vi "FlexMag - 23-03-2023.vi"() -> ()   [LabVIEW 2018] (continued)
          tunnel: [w8156 w8268 w8304 w8346 w8389 w8424 w8458 w8492] -> w8125
          frame 0, Default {
            n4720 = stacked-sequence {
              seq-local: [w8166 _] -> [_ w8224]
              seq-local: [w8165 _] -> [_ w8222]
              tunnel: w8159 -> [w8175 _]
              tunnel: w8158 -> [w8174 _]
              tunnel: [_ w8226] -> w8157
              tunnel: [_ w8225] -> w8156
              frame #0 {
                # "Address"
                # "Address"
                n4721 = Concatenate Strings("002" ("write buffer"), "00" ("string"), "309" ("string"), "02" ("string"), "=?" ("string")) -> (w8184:string)
                n4722 = String To Byte Array(string=w8184) -> (unsigned byte array=w8189:u8[])
                n4723 = for {
                  tunnel: w8189 -> [w8221] mode=indexing
                  shift-right: [w8219] -> w8191
                  shift-left: u8 0 -> [w8220]
                  n4724 = Add(x=w8221, y=w8220) -> (x+y=w8219:u8)
                }
                n4725 = Number To Decimal String(number=w8191) -> (decimal integer string=w8186:string)  [unwired: 1 in]
                n4726 = String Length(string=w8186) -> (length=w8187:i32)
                n4727 = case shown="3" w8187 {
                  tunnel: w8186 -> [_ w8214 w8217 w8218]
                  tunnel: ["" w8212 w8215 w8218] -> w8185
                  frame 0, Default {
                  }
                  frame 1 {
                    n4728 = Concatenate Strings("00" ("string"), w8214) -> (w8212:string)
                  }
                  frame 2 {
                    n4729 = Concatenate Strings("0" ("string"), w8217) -> (w8215:string)
                  }
                  frame 3 {
                  }
                }
                n4730 = Concatenate Strings(w8184, w8185, "\r") -> (w8176:string)
                n4731 = VISA Write(VISA resource name=w8175, write buffer=w8176, error in (no error)=w8174) -> (VISA resource name out=w8179:refnum<visa-resource-name>, error out=w8178:errorcluster)  [unwired: 1 out]
                n4732 = stacked-sequence {
                  tunnel: [w8210] -> w8181
                  tunnel: w8179 -> [w8210]
                  tunnel: [w8209] -> w8180
                  tunnel: w8178 -> [w8209]
                  frame #0 {
                    n4733 = Wait (ms)(milliseconds to wait=u32 100) -> ()  [unwired: 1 out]
                  }
                }
                n4734 = property class="Instr"(reference=w8181, error in=w8180) -> (reference out=w8183:refnum<visa-resource-name>, error out=w8182:errorcluster, "Serial Settings:Number of Bytes at Serial Port"=w8177:u32)
                n4735 = VISA Read(VISA resource name=w8183, byte count=w8177, error in (no error)=w8182) -> (VISA resource name out=w8166:refnum<visa-resource-name>, read buffer=w8160:string, error out=w8165:errorcluster)  [unwired: 1 out]
                n4736 = String Length(string=w8160) -> (length=w8173:i32)
                n4737 = Not Equal To 0?(x=w8173) -> (x != 0?=w8164:bool)
                n4738 = feedback #142() -> (w8162:bool)  [unwired: 1 in]
                n4739 = Concatenate Strings("002" ("regular expression"), "1030906" ("regular expression")) -> (w8172:string)
                n4740 = case shown="False" w8164 {
                  tunnel: [FALSE w8201] -> w8161
                  tunnel: [TRUE FALSE] -> w8163
                  tunnel: w8162 -> [_ w8199]
                  frame False {
                  }
                  frame True {
                    n4741 = call "Elapsed Time37"("Reset"=w8199) -> ("Elapsed Time (s)"=w8202:dbl)  [unwired: 11 in, 7 out]
                    n4742 = Greater?(x=w8202, y=5.0) -> (0:w8201:bool)
                  }
                }
                "tp1 com" <- w8161
                n4743 = feedback-in #142(w8163) -> ()
                n4744 = Match Pattern(string=w8160, regular expression=w8172) -> (after substring=w8167:string)  [unwired: 4 out]
                n4745 = String Length(string=w8167) -> (length=w8169:i32)
                n4746 = Not Equal To 0?(x=w8169) -> (x != 0?=w8168:bool)
                n4747 = case shown="True" w8168 {
                  tunnel: w8167 -> [_ w8204]
                  frame False {
                  }
                  frame True {
                    n4748 = String Subset(string=w8204, length (rest)=6 ("length (rest)")) -> (substring=w8206:string)  [unwired: 1 out]
                    n4749 = Decimal String To Number(string=w8206) -> (number=→"Tp1 speed gui":i32)  [unwired: 3 out]
                    "tp1 readout" <- w8204
                  }
                }
              }
              frame #1 {
                # "Address"
                # "Address"
                n4750 = Concatenate Strings("002" ("write buffer"), "00" ("string"), "307" ("string"), "02" ("string"), "=?" ("string")) -> (w8239:string)
                n4751 = String To Byte Array(string=w8239) -> (unsigned byte array=w8244:u8[])
                n4752 = for {
                  tunnel: w8244 -> [w8265] mode=indexing
                  shift-right: [w8263] -> w8246
                  shift-left: u8 0 -> [w8264]
                  n4753 = Add(x=w8265, y=w8264) -> (x+y=w8263:u8)
                }
                n4754 = Number To Decimal String(number=w8246) -> (decimal integer string=w8241:string)  [unwired: 1 in]
                n4755 = String Length(string=w8241) -> (length=w8242:i32)
                n4756 = case shown="0, Default" w8242 {
                  tunnel: w8241 -> [_ w8258 w8261 w8262]
                  tunnel: ["" w8256 w8259 w8262] -> w8240
                  frame 0, Default {
                  }
                  frame 1 {
                    n4757 = Concatenate Strings("00" ("string"), w8258) -> (w8256:string)
                  }
                  frame 2 {
                    n4758 = Concatenate Strings("0" ("string"), w8261) -> (w8259:string)
                  }
                  frame 3 {
                  }
                }
                n4759 = Concatenate Strings(w8239, w8240, "\r") -> (w8231:string)
                n4760 = VISA Write(VISA resource name=w8224, write buffer=w8231, error in (no error)=w8222) -> (VISA resource name out=w8234:refnum<visa-resource-name>, error out=w8233:errorcluster)  [unwired: 1 out]
                n4761 = stacked-sequence {
                  tunnel: [w8254] -> w8236
                  tunnel: w8234 -> [w8254]
                  tunnel: [w8253] -> w8235
                  tunnel: w8233 -> [w8253]
                  frame #0 {
                    n4762 = Wait (ms)(milliseconds to wait=u32 100) -> ()  [unwired: 1 out]
                  }
                }
                n4763 = property class="Instr"(reference=w8236, error in=w8235) -> (reference out=w8238:refnum<visa-resource-name>, error out=w8237:errorcluster, "Serial Settings:Number of Bytes at Serial Port"=w8232:u32)
                n4764 = VISA Read(VISA resource name=w8238, byte count=w8232, error in (no error)=w8237) -> (VISA resource name out=w8226:refnum<visa-resource-name>, read buffer=w8230:string, error out=w8225:errorcluster)  [unwired: 1 out]
                n4765 = Concatenate Strings("002" ("regular expression"), "1030706" ("regular expression")) -> (w8229:string)
                n4766 = Match Pattern(string=w8230, regular expression=w8229) -> (after substring=→"after substring":string)  [unwired: 4 out]
              }
            }
          }
          frame 1 {
            # "Cheksum 3 haneli olmalı"
            # "Address"
            n4767 = Concatenate Strings("002" ("write buffer"), "10" ("string"), "010" ("string"), "06" ("string"), "111111" ("string")) -> (w8275:string)
            n4768 = String To Byte Array(string=w8275) -> (unsigned byte array=w8280:u8[])
            n4769 = for {
              tunnel: w8280 -> [w8301] mode=indexing
              shift-right: [w8299] -> w8282
              shift-left: u8 0 -> [w8300]
              n4770 = Add(x=w8301, y=w8300) -> (x+y=w8299:u8)
            }
            n4771 = Number To Decimal String(number=w8282) -> (decimal integer string=w8277:string)  [unwired: 1 in]
            n4772 = String Length(string=w8277) -> (length=w8278:i32)
            n4773 = local write "Tp1 auto start"(FALSE ("Tp1_auto_start")) -> ()
            n4774 = case shown="1" w8278 {
              tunnel: w8277 -> [_ w8294 w8297 w8298]
              tunnel: ["" w8292 w8295 w8298] -> w8276
              frame 0, Default {
              }
              frame 1 {
                n4775 = Concatenate Strings("00" ("string"), w8294) -> (w8292:string)
              }
              frame 2 {
                n4776 = Concatenate Strings("0" ("string"), w8297) -> (w8295:string)
              }
              frame 3 {
              }
            }
            n4777 = local write "Tp1_stop_cmnd"(FALSE ("Tp1_stop_cmnd")) -> ()
            n4778 = Concatenate Strings(w8275, w8276, "\r") -> (w8272:string)
            n4779 = VISA Write(VISA resource name=w8271, write buffer=w8272, error in (no error)=w8270) -> (VISA resource name out=w8274:refnum<visa-resource-name>, error out=w8273:errorcluster)  [unwired: 1 out]
            n4780 = stacked-sequence {
              tunnel: [w8290] -> w8269
              tunnel: w8274 -> [w8290]
              tunnel: [w8289] -> w8268
              tunnel: w8273 -> [w8289]
              frame #0 {
                n4781 = Wait (ms)(milliseconds to wait=u32 100) -> ()  [unwired: 1 out]
              }
            }
          }
          frame 2 {
            # "Cheksum 3 haneli olmalı"
            # "Address"
            n4782 = Concatenate Strings("002" ("write buffer"), "10" ("string"), "010" ("string"), "06" ("string"), "000000" ("string")) -> (w8311:string)
            n4783 = String To Byte Array(string=w8311) -> (unsigned byte array=w8316:u8[])
            n4784 = for {
              tunnel: w8316 -> [w8337] mode=indexing
              shift-right: [w8335] -> w8318
              shift-left: u8 0 -> [w8336]
              n4785 = Add(x=w8337, y=w8336) -> (x+y=w8335:u8)
            }
            n4786 = Number To Decimal String(number=w8318) -> (decimal integer string=w8313:string)  [unwired: 1 in]
            n4787 = local write "Tp1 auto stop"(FALSE ("Tp1_auto_stop")) -> ()
            n4788 = String Length(string=w8313) -> (length=w8314:i32)
            n4789 = case shown="0, Default" w8314 {
              tunnel: w8313 -> [_ w8330 w8333 w8334]
              tunnel: ["" w8328 w8331 w8334] -> w8312
              frame 0, Default {
              }
              frame 1 {
                n4790 = Concatenate Strings("00" ("string"), w8330) -> (w8328:string)
              }
              frame 2 {
                n4791 = Concatenate Strings("0" ("string"), w8333) -> (w8331:string)
              }
              frame 3 {
              }
            }
            n4792 = Concatenate Strings(w8311, w8312, "\r") -> (w8308:string)
            n4793 = VISA Write(VISA resource name=w8307, write buffer=w8308, error in (no error)=w8306) -> (VISA resource name out=w8310:refnum<visa-resource-name>, error out=w8309:errorcluster)  [unwired: 1 out]
            n4794 = stacked-sequence {
              tunnel: [w8326] -> w8305
              tunnel: w8310 -> [w8326]
              tunnel: [w8325] -> w8304
              tunnel: w8309 -> [w8325]
              frame #0 {
                n4795 = Wait (ms)(milliseconds to wait=u32 100) -> ()  [unwired: 1 out]
              }
            }
            "Tp1_stop_cmnd" <- TRUE ("Tp_stop_cmnd")
          }
          frame 3 {
            # "Cheksum 3 haneli olmalı"
            # "Address"
            n4796 = Multiply(x="Low_speed_value", y=ext 10.0) -> (x*y=w8343:ext)
            n4797 = To Unsigned Long Integer(number=w8343) -> (unsigned 32bit integer=w8342:u32)
            n4798 = Number To Decimal String(number=w8342) -> (decimal integer string=w8340:string)  [unwired: 1 out]
            n4799 = String Length(string=w8340) -> (length=w8341:i32)
            n4800 = case shown="0, Default" w8341 {
              tunnel: w8340 -> [_ w8369 w8372 w8373]
              tunnel: ["" w8368 w8371 w8373] -> w8339
              frame 0, Default {
              }
              frame 1 {
                n4801 = Concatenate Strings(w8369, "00" ("string")) -> (w8368:string)
              }
              frame 2 {
                n4802 = Concatenate Strings(w8372, "0" ("string")) -> (w8371:string)
              }
              frame 3 {
              }
            }
            n4803 = Concatenate Strings("002" ("write buffer"), "10" ("string"), "707" ("string"), "06" ("string"), "00" ("string"), w8339) -> (w8353:string)
            n4804 = String To Byte Array(string=w8353) -> (unsigned byte array=w8358:u8[])
            n4805 = for {
              tunnel: w8358 -> [w8387] mode=indexing
              shift-right: [w8385] -> w8360
              shift-left: u8 0 -> [w8386]
              n4806 = Add(x=w8387, y=w8386) -> (x+y=w8385:u8)
            }
            n4807 = Number To Decimal String(number=w8360) -> (decimal integer string=w8355:string)  [unwired: 1 in]
            n4808 = String Length(string=w8355) -> (length=w8356:i32)
            n4809 = case shown="3" w8356 {
              tunnel: w8355 -> [_ w8380 w8383 w8384]
              tunnel: ["" w8378 w8381 w8384] -> w8354
              frame 0, Default {
              }
              frame 1 {
                n4810 = Concatenate Strings("00" ("string"), w8380) -> (w8378:string)
              }
              frame 2 {
                n4811 = Concatenate Strings("0" ("string"), w8383) -> (w8381:string)
              }
              frame 3 {
              }
            }
            n4812 = local write "Tp1 auto set speed"(FALSE ("Tp1_auto_set_speed")) -> ()
            n4813 = Concatenate Strings(w8353, w8354, "\r") -> (w8350:string)
            n4814 = VISA Write(VISA resource name=w8349, write buffer=w8350, error in (no error)=w8348) -> (VISA resource name out=w8352:refnum<visa-resource-name>, error out=w8351:errorcluster)  [unwired: 1 out]
            n4815 = stacked-sequence {
              tunnel: [w8376] -> w8347
              tunnel: w8352 -> [w8376]
              tunnel: [w8375] -> w8346
              tunnel: w8351 -> [w8375]
              frame #0 {
                n4816 = Wait (ms)(milliseconds to wait=u32 100) -> ()  [unwired: 1 out]
              }
            }
          }
          frame 4 {
            # "Cheksum 3 haneli olmalı"
            # "Address"
            n4817 = Concatenate Strings("002" ("write buffer"), "10" ("string"), "026" ("string"), "03" ("string"), "001" ("string")) -> (w8396:string)
            n4818 = String To Byte Array(string=w8396) -> (unsigned byte array=w8401:u8[])
            n4819 = for {
              tunnel: w8401 -> [w8422] mode=indexing
              shift-right: [w8420] -> w8403
              shift-left: u8 0 -> [w8421]
              n4820 = Add(x=w8422, y=w8421) -> (x+y=w8420:u8)
            }
            n4821 = Number To Decimal String(number=w8403) -> (decimal integer string=w8398:string)  [unwired: 1 in]
            n4822 = local write "Tp1 auto low speed"(FALSE) -> ()
            n4823 = String Length(string=w8398) -> (length=w8399:i32)
            n4824 = case shown="0, Default" w8399 {
              tunnel: w8398 -> [_ w8415 w8418 w8419]
              tunnel: ["" w8413 w8416 w8419] -> w8397
              frame 0, Default {
              }
              frame 1 {
                n4825 = Concatenate Strings("00" ("string"), w8415) -> (w8413:string)
              }
              frame 2 {
                n4826 = Concatenate Strings("0" ("string"), w8418) -> (w8416:string)
              }
              frame 3 {
              }
            }
            n4827 = Concatenate Strings(w8396, w8397, "\r") -> (w8393:string)
            n4828 = VISA Write(VISA resource name=w8392, write buffer=w8393, error in (no error)=w8391) -> (VISA resource name out=w8395:refnum<visa-resource-name>, error out=w8394:errorcluster)  [unwired: 1 out]
            n4829 = stacked-sequence {
              tunnel: [w8411] -> w8390
              tunnel: w8395 -> [w8411]
              tunnel: [w8410] -> w8389
              tunnel: w8394 -> [w8410]
              frame #0 {
                n4830 = Wait (ms)(milliseconds to wait=u32 100) -> ()  [unwired: 1 out]
              }
            }
          }
          frame 5 {
            # "Cheksum 3 haneli olmalı"
            # "Address"
            n4831 = Concatenate Strings("002" ("write buffer"), "10" ("string"), "026" ("string"), "03" ("string"), "000" ("string")) -> (w8431:string)
            n4832 = String To Byte Array(string=w8431) -> (unsigned byte array=w8436:u8[])
            n4833 = for {
              tunnel: w8436 -> [w8457] mode=indexing
              shift-right: [w8455] -> w8438
              shift-left: u8 0 -> [w8456]
              n4834 = Add(x=w8457, y=w8456) -> (x+y=w8455:u8)
            }
            n4835 = Number To Decimal String(number=w8438) -> (decimal integer string=w8433:string)  [unwired: 1 in]
            n4836 = String Length(string=w8433) -> (length=w8434:i32)
            n4837 = case shown="0, Default" w8434 {
              tunnel: w8433 -> [_ w8450 w8453 w8454]
              tunnel: ["" w8448 w8451 w8454] -> w8432
              frame 0, Default {
              }
              frame 1 {
                n4838 = Concatenate Strings("00" ("string"), w8450) -> (w8448:string)
              }
              frame 2 {
                n4839 = Concatenate Strings("0" ("string"), w8453) -> (w8451:string)
              }
              frame 3 {
              }
            }
            n4840 = local write "Tp1 auto normal speed"(FALSE ("Tp1_auto_normal_speed")) -> ()
            n4841 = Concatenate Strings(w8431, w8432, "\r") -> (w8428:string)
            n4842 = VISA Write(VISA resource name=w8427, write buffer=w8428, error in (no error)=w8426) -> (VISA resource name out=w8430:refnum<visa-resource-name>, error out=w8429:errorcluster)  [unwired: 1 out]
            n4843 = stacked-sequence {
              tunnel: [w8446] -> w8425
              tunnel: w8430 -> [w8446]
              tunnel: [w8445] -> w8424
              tunnel: w8429 -> [w8445]
              frame #0 {
                n4844 = Wait (ms)(milliseconds to wait=u32 100) -> ()  [unwired: 1 out]
              }
            }
          }
          frame 6 {
            # "Cheksum 3 haneli olmalı"
            # "Address"
            n4845 = Concatenate Strings("002" ("write buffer"), "10" ("string"), "023" ("string"), "06" ("string"), "111111" ("string")) -> (w8465:string)
            n4846 = String To Byte Array(string=w8465) -> (unsigned byte array=w8470:u8[])
            n4847 = for {
              tunnel: w8470 -> [w8491] mode=indexing
              shift-right: [w8489] -> w8472
              shift-left: u8 0 -> [w8490]
              n4848 = Add(x=w8491, y=w8490) -> (x+y=w8489:u8)
            }
            n4849 = Number To Decimal String(number=w8472) -> (decimal integer string=w8467:string)  [unwired: 1 in]
            n4850 = String Length(string=w8467) -> (length=w8468:i32)
            n4851 = case shown="0, Default" w8468 {
              tunnel: w8467 -> [_ w8484 w8487 w8488]
              tunnel: ["" w8482 w8485 w8488] -> w8466
              frame 0, Default {
              }
              frame 1 {
                n4852 = Concatenate Strings("00" ("string"), w8484) -> (w8482:string)
              }
              frame 2 {
                n4853 = Concatenate Strings("0" ("string"), w8487) -> (w8485:string)
              }
              frame 3 {
              }
            }
            n4854 = Concatenate Strings(w8465, w8466, "\r") -> (w8462:string)
            n4855 = VISA Write(VISA resource name=w8461, write buffer=w8462, error in (no error)=w8460) -> (VISA resource name out=w8464:refnum<visa-resource-name>, error out=w8463:errorcluster)  [unwired: 1 out]
            n4856 = stacked-sequence {
              tunnel: [w8480] -> w8459
              tunnel: w8464 -> [w8480]
              tunnel: [w8479] -> w8458
              tunnel: w8463 -> [w8479]
              frame #0 {
                n4857 = Wait (ms)(milliseconds to wait=u32 100) -> ()  [unwired: 1 out]
              }
            }
          }
          frame 7 {
            # "Cheksum 3 haneli olmalı"
            # "Address"
            n4858 = Concatenate Strings("002" ("write buffer"), "10" ("string"), "023" ("string"), "06" ("string"), "000000" ("string")) -> (w8499:string)
            n4859 = String To Byte Array(string=w8499) -> (unsigned byte array=w8504:u8[])
            n4860 = for {
              tunnel: w8504 -> [w8525] mode=indexing
              shift-right: [w8523] -> w8506
              shift-left: u8 0 -> [w8524]
              n4861 = Add(x=w8525, y=w8524) -> (x+y=w8523:u8)
            }
            n4862 = Number To Decimal String(number=w8506) -> (decimal integer string=w8501:string)  [unwired: 1 in]
            n4863 = String Length(string=w8501) -> (length=w8502:i32)
            n4864 = case shown="0, Default" w8502 {
              tunnel: w8501 -> [_ w8518 w8521 w8522]
              tunnel: ["" w8516 w8519 w8522] -> w8500
              frame 0, Default {
              }
              frame 1 {
                n4865 = Concatenate Strings("00" ("string"), w8518) -> (w8516:string)
              }
              frame 2 {
                n4866 = Concatenate Strings("0" ("string"), w8521) -> (w8519:string)
              }
              frame 3 {
              }
            }
            n4867 = Concatenate Strings(w8499, w8500, "\r") -> (w8496:string)
            n4868 = VISA Write(VISA resource name=w8495, write buffer=w8496, error in (no error)=w8494) -> (VISA resource name out=w8498:refnum<visa-resource-name>, error out=w8497:errorcluster)  [unwired: 1 out]
            n4869 = stacked-sequence {
              tunnel: [w8514] -> w8493
              tunnel: w8498 -> [w8514]
              tunnel: [w8513] -> w8492
              tunnel: w8497 -> [w8513]
              frame #0 {
                n4870 = Wait (ms)(milliseconds to wait=u32 100) -> ()  [unwired: 1 out]
              }
            }
          }
        }
      }
      frame #1 {
        n4871 = Compound Arithmetic op=OR("Tp2 start gui", "Tp2 start gui 1", "Tp2 auto start") -> (w8530:bool)
        n4872 = Or(x="Tp2 low speed gui", y="Tp2 auto low speed") -> (x .or. y?=w8545:bool)
        n4873 = Or(x="Tp2 normal speed gui", y="Tp2 auto normal speed") -> (x .or. y?=w8540:bool)
        n4874 = Compound Arithmetic op=OR("Tp2 stop gui", "Tp2 stop gui 1", "Tp2 auto stop") -> (w8532:bool)
        n4875 = Or(x="Tp2 set speed gui", y="Tp2 auto set speed") -> (x .or. y?=w8546:bool)
        n4876 = case shown="True" w8530 {
          tunnel: [FALSE w8556] -> w8529
          frame False {
          }
          frame True {
            n4877 = case shown="False" "tp2 start safety" {
              tunnel: [FALSE TRUE] -> w8556
              frame False {
                n4878 = local write "Tp2 auto start"(FALSE ("Tp1_auto_start")) -> ()
                n4879 = local write "Warning Message"("CH2 TP cannot be started." ("Error Message")) -> ()
              }
              frame True {
              }
            }
          }
        }
        n4880 = Build Array(FALSE, w8529, w8532, w8546, w8545, w8540, "Tp2 start initial", "Tp2 stop initial") -> (w8552:bool[])
        n4881 = Boolean Array To Number(Boolean array=w8552) -> (number=w8553:u32)
        n4882 = Mantissa & Exponent(0:w8553) -> (2:w8550:dbl)  [unwired: 1 out]
        n4883 = case shown="0, Default" w8550 {
          tunnel: w8549 -> [w8561 w8676 w8712 w8754 w8797 w8832 w8866 w8900]
          tunnel: w8531 -> [w8562 w8675 w8711 w8753 w8796 w8831 w8865 w8899]
          tunnel: [w8564 w8674 w8710 w8752 w8795 w8830 w8864 w8898] -> w8527
          tunnel: [w8563 w8673 w8709 w8751 w8794 w8829 w8863 w8897] -> w8526
          frame 0, Default {
            n4884 = stacked-sequence {
              seq-local: [w8570 _] -> [_ w8628]
              seq-local: [w8569 _] -> [_ w8629]
              tunnel: w8561 -> [w8580 _]
              tunnel: w8562 -> [w8579 _]
              tunnel: [_ w8631] -> w8564
              tunnel: [_ w8630] -> w8563
              frame #0 {
                # "Address"
                # "Cheksum 3 haneli olmalı"
                # "Address"
                n4885 = Concatenate Strings("001" ("write buffer"), "00" ("string"), "309" ("string"), "02" ("string"), "=?" ("string")) -> (w8589:string)
                n4886 = String To Byte Array(string=w8589) -> (unsigned byte array=w8594:u8[])
                n4887 = for {
                  tunnel: w8594 -> [w8626] mode=indexing
                  shift-right: [w8624] -> w8596
                  shift-left: u8 0 -> [w8625]
                  n4888 = Add(x=w8626, y=w8625) -> (x+y=w8624:u8)
                }
                n4889 = Number To Decimal String(number=w8596) -> (decimal integer string=w8591:string)  [unwired: 1 in]
                n4890 = String Length(string=w8591) -> (length=w8592:i32)
                n4891 = case shown="0, Default" w8592 {
                  tunnel: w8591 -> [_ w8619 w8622 w8623]
                  tunnel: ["" w8617 w8620 w8623] -> w8590
                  frame 0, Default {
                  }
                  frame 1 {
                    n4892 = Concatenate Strings("00" ("string"), w8619) -> (w8617:string)
                  }
                  frame 2 {
                    n4893 = Concatenate Strings("0" ("string"), w8622) -> (w8620:string)
                  }
                  frame 3 {
                  }
                }
                n4894 = Concatenate Strings(w8589, w8590, "\r") -> (w8581:string)
                n4895 = VISA Write(VISA resource name=w8580, write buffer=w8581, error in (no error)=w8579) -> (VISA resource name out=w8584:refnum<visa-resource-name>, error out=w8583:errorcluster)  [unwired: 1 out]
                n4896 = stacked-sequence {
                  tunnel: [w8615] -> w8586
                  tunnel: w8584 -> [w8615]
                  tunnel: [w8614] -> w8585
                  tunnel: w8583 -> [w8614]
                  frame #0 {
                    n4897 = Wait (ms)(milliseconds to wait=u32 100) -> ()  [unwired: 1 out]
                  }
                }
                n4898 = property class="Instr"(reference=w8586, error in=w8585) -> (reference out=w8588:refnum<visa-resource-name>, error out=w8587:errorcluster, "Serial Settings:Number of Bytes at Serial Port"=w8582:u32)
                n4899 = VISA Read(VISA resource name=w8588, byte count=w8582, error in (no error)=w8587) -> (VISA resource name out=w8570:refnum<visa-resource-name>, read buffer=w8577:string, error out=w8569:errorcluster)  [unwired: 1 out]
                n4900 = String Length(string=w8577) -> (length=w8578:i32)
                n4901 = Not Equal To 0?(x=w8578) -> (x != 0?=w8566:bool)
                n4902 = Concatenate Strings("001" ("regular expression"), "1030906" ("regular expression")) -> (w8576:string)
                n4903 = Match Pattern(string=w8577, regular expression=w8576) -> (after substring=w8571:string)  [unwired: 4 out]
                n4904 = feedback #143() -> (w8567:bool)  [unwired: 1 in]
                n4905 = String Length(string=w8571) -> (length=w8573:i32)
                n4906 = Not Equal To 0?(x=w8573) -> (x != 0?=w8572:bool)
                n4907 = case shown="False" w8566 {
                  tunnel: [FALSE w8606] -> w8565
                  tunnel: [TRUE FALSE] -> w8568
                  tunnel: w8567 -> [_ w8604]
                  frame False {
                  }
                  frame True {
                    n4908 = call "Elapsed Time38"("Reset"=w8604) -> ("Elapsed Time (s)"=w8607:dbl)  [unwired: 11 in, 7 out]
                    n4909 = Greater?(x=w8607, y=5.0) -> (0:w8606:bool)
                  }
                }
                "tp2 com" <- w8565
                n4910 = feedback-in #143(w8568) -> ()
                n4911 = case shown="True" w8572 {
                  tunnel: w8571 -> [_ w8609]
                  frame False {
                  }
                  frame True {
                    n4912 = String Subset(string=w8609, length (rest)=6 ("length (rest)")) -> (substring=w8611:string)  [unwired: 1 out]
                    n4913 = Decimal String To Number(string=w8611) -> (number=→"Tp2 speed gui":i32)  [unwired: 3 out]
                    "tp2 readout" <- w8609
                  }
                }
              }
              frame #1 {
                # "Address"
                # "Cheksum 3 haneli olmalı"
                # "Address"
                n4914 = Concatenate Strings("001" ("write buffer"), "00" ("string"), "307" ("string"), "02" ("string"), "=?" ("string")) -> (w8644:string)
                n4915 = String To Byte Array(string=w8644) -> (unsigned byte array=w8649:u8[])
                n4916 = for {
                  tunnel: w8649 -> [w8670] mode=indexing
                  shift-right: [w8668] -> w8651
                  shift-left: u8 0 -> [w8669]
                  n4917 = Add(x=w8670, y=w8669) -> (x+y=w8668:u8)
                }
                n4918 = Number To Decimal String(number=w8651) -> (decimal integer string=w8646:string)  [unwired: 1 in]
                n4919 = String Length(string=w8646) -> (length=w8647:i32)
                n4920 = case shown="0, Default" w8647 {
                  tunnel: w8646 -> [_ w8663 w8666 w8667]
                  tunnel: ["" w8661 w8664 w8667] -> w8645
                  frame 0, Default {
                  }
                  frame 1 {
                    n4921 = Concatenate Strings("00" ("string"), w8663) -> (w8661:string)
                  }
                  frame 2 {
                    n4922 = Concatenate Strings("0" ("string"), w8666) -> (w8664:string)
                  }
                  frame 3 {
                  }
                }
                n4923 = Concatenate Strings(w8644, w8645, "\r") -> (w8636:string)
                n4924 = VISA Write(VISA resource name=w8628, write buffer=w8636, error in (no error)=w8629) -> (VISA resource name out=w8639:refnum<visa-resource-name>, error out=w8638:errorcluster)  [unwired: 1 out]
                n4925 = stacked-sequence {
                  tunnel: [w8659] -> w8641
                  tunnel: w8639 -> [w8659]
                  tunnel: [w8658] -> w8640
                  tunnel: w8638 -> [w8658]
                  frame #0 {
                    n4926 = Wait (ms)(milliseconds to wait=u32 100) -> ()  [unwired: 1 out]
                  }
                }
                n4927 = property class="Instr"(reference=w8641, error in=w8640) -> (reference out=w8643:refnum<visa-resource-name>, error out=w8642:errorcluster, "Serial Settings:Number of Bytes at Serial Port"=w8637:u32)
                n4928 = VISA Read(VISA resource name=w8643, byte count=w8637, error in (no error)=w8642) -> (VISA resource name out=w8631:refnum<visa-resource-name>, read buffer=w8635:string, error out=w8630:errorcluster)  [unwired: 1 out]
                n4929 = Concatenate Strings("001" ("regular expression"), "1030706" ("regular expression")) -> (w8634:string)
                n4930 = Match Pattern(string=w8635, regular expression=w8634) -> (after substring=→"after substring 2":string)  [unwired: 4 out]
              }
            }
          }
          frame 1 {
            # "Cheksum 3 haneli olmalı"
            # "Address"
            n4931 = Concatenate Strings("001" ("write buffer"), "10" ("string"), "010" ("string"), "06" ("string"), "111111" ("string")) -> (w8680:string)
            n4932 = String To Byte Array(string=w8680) -> (unsigned byte array=w8685:u8[])
            n4933 = for {
              tunnel: w8685 -> [w8706] mode=indexing
              shift-right: [w8704] -> w8687
              shift-left: u8 0 -> [w8705]
              n4934 = Add(x=w8706, y=w8705) -> (x+y=w8704:u8)
            }
            n4935 = local write "Tp2 auto start"(FALSE ("Tp2_auto_start")) -> ()
            n4936 = Number To Decimal String(number=w8687) -> (decimal integer string=w8682:string)  [unwired: 1 in]
            n4937 = String Length(string=w8682) -> (length=w8683:i32)
            n4938 = case shown="0, Default" w8683 {
              tunnel: w8682 -> [_ w8699 w8702 w8703]
              tunnel: ["" w8697 w8700 w8703] -> w8681
              frame 0, Default {
              }
              frame 1 {
                n4939 = Concatenate Strings("00" ("string"), w8699) -> (w8697:string)
              }
              frame 2 {
                n4940 = Concatenate Strings("0" ("string"), w8702) -> (w8700:string)
              }
              frame 3 {
              }
            }
            n4941 = Concatenate Strings(w8680, w8681, "\r") -> (w8677:string)
            n4942 = local write "Tp2_stop_cmnd"(FALSE ("Tp2_stop_cmnd")) -> ()
            n4943 = VISA Write(VISA resource name=w8676, write buffer=w8677, error in (no error)=w8675) -> (VISA resource name out=w8679:refnum<visa-resource-name>, error out=w8678:errorcluster)  [unwired: 1 out]
            n4944 = stacked-sequence {
              tunnel: [w8695] -> w8674
              tunnel: w8679 -> [w8695]
              tunnel: [w8694] -> w8673
              tunnel: w8678 -> [w8694]
              frame #0 {
                n4945 = Wait (ms)(milliseconds to wait=u32 100) -> ()  [unwired: 1 out]
              }
            }
          }
          frame 2 {
            # "Cheksum 3 haneli olmalı"
            # "Address"
            n4946 = Concatenate Strings("001" ("write buffer"), "10" ("string"), "010" ("string"), "06" ("string"), "000000" ("string")) -> (w8716:string)
            n4947 = String To Byte Array(string=w8716) -> (unsigned byte array=w8721:u8[])
            n4948 = for {
              tunnel: w8721 -> [w8742] mode=indexing
              shift-right: [w8740] -> w8723
              shift-left: u8 0 -> [w8741]
              n4949 = Add(x=w8742, y=w8741) -> (x+y=w8740:u8)
            }
            n4950 = local write "Tp2 auto stop"(FALSE ("Tp2_auto_stop")) -> ()
            n4951 = Number To Decimal String(number=w8723) -> (decimal integer string=w8718:string)  [unwired: 1 in]
            n4952 = String Length(string=w8718) -> (length=w8719:i32)
            n4953 = case shown="0, Default" w8719 {
              tunnel: w8718 -> [_ w8735 w8738 w8739]
              tunnel: ["" w8733 w8736 w8739] -> w8717
              frame 0, Default {
              }
              frame 1 {
                n4954 = Concatenate Strings("00" ("string"), w8735) -> (w8733:string)
              }
              frame 2 {
                n4955 = Concatenate Strings("0" ("string"), w8738) -> (w8736:string)
              }
              frame 3 {
              }
            }
            n4956 = Concatenate Strings(w8716, w8717, "\r") -> (w8713:string)
            n4957 = VISA Write(VISA resource name=w8712, write buffer=w8713, error in (no error)=w8711) -> (VISA resource name out=w8715:refnum<visa-resource-name>, error out=w8714:errorcluster)  [unwired: 1 out]
            n4958 = stacked-sequence {
              tunnel: [w8731] -> w8710
              tunnel: w8715 -> [w8731]
              tunnel: [w8730] -> w8709
              tunnel: w8714 -> [w8730]
              frame #0 {
                n4959 = Wait (ms)(milliseconds to wait=u32 100) -> ()  [unwired: 1 out]
              }
            }
            "Tp2_stop_cmnd" <- TRUE ("Tp2_stop_cmnd")
          }
          frame 3 {
            # "Cheksum 3 haneli olmalı"
            # "Address"
            n4960 = Multiply(x="Low_speed_value 2", y=ext 10.0) -> (x*y=w8748:ext)
            n4961 = To Unsigned Long Integer(number=w8748) -> (unsigned 32bit integer=w8747:u32)
            n4962 = Number To Decimal String(number=w8747) -> (decimal integer string=w8745:string)  [unwired: 1 out]
            n4963 = String Length(string=w8745) -> (length=w8746:i32)
            n4964 = case shown="3" w8746 {
              tunnel: w8745 -> [_ w8774 w8777 w8778]
              tunnel: ["" w8773 w8776 w8778] -> w8744
              frame 0, Default {
              }
              frame 1 {
                n4965 = Concatenate Strings(w8774, "00" ("string")) -> (w8773:string)
              }
              frame 2 {
                n4966 = Concatenate Strings(w8777, "0" ("string")) -> (w8776:string)
              }
              frame 3 {
              }
            }
            n4967 = Concatenate Strings("001" ("write buffer"), "10" ("string"), "707" ("string"), "06" ("string"), "00" ("string"), w8744) -> (w8758:string)
            n4968 = String To Byte Array(string=w8758) -> (unsigned byte array=w8763:u8[])
            n4969 = for {
              tunnel: w8763 -> [w8792] mode=indexing
              shift-right: [w8790] -> w8765
              shift-left: u8 0 -> [w8791]
              n4970 = Add(x=w8792, y=w8791) -> (x+y=w8790:u8)
            }
            n4971 = Number To Decimal String(number=w8765) -> (decimal integer string=w8760:string)  [unwired: 1 in]
            n4972 = String Length(string=w8760) -> (length=w8761:i32)
            n4973 = case shown="0, Default" w8761 {
              tunnel: w8760 -> [_ w8785 w8788 w8789]
              tunnel: ["" w8783 w8786 w8789] -> w8759
              frame 0, Default {
              }
              frame 1 {
                n4974 = Concatenate Strings("00" ("string"), w8785) -> (w8783:string)
              }
              frame 2 {
                n4975 = Concatenate Strings("0" ("string"), w8788) -> (w8786:string)
              }
              frame 3 {
              }
            }
            n4976 = Concatenate Strings(w8758, w8759, "\r") -> (w8755:string)
            n4977 = VISA Write(VISA resource name=w8754, write buffer=w8755, error in (no error)=w8753) -> (VISA resource name out=w8757:refnum<visa-resource-name>, error out=w8756:errorcluster)  [unwired: 1 out]
            n4978 = stacked-sequence {
              tunnel: [w8781] -> w8752
              tunnel: w8757 -> [w8781]
              tunnel: [w8780] -> w8751
              tunnel: w8756 -> [w8780]
              frame #0 {
                n4979 = Wait (ms)(milliseconds to wait=u32 100) -> ()  [unwired: 1 out]
              }
            }
            n4980 = local write "Tp2 auto set speed"(FALSE ("Tp2_auto_set_speed")) -> ()
          }
          frame 4 {
            # "Cheksum 3 haneli olmalı"
            # "Address"
            n4981 = Concatenate Strings("001" ("write buffer"), "10" ("string"), "026" ("string"), "03" ("string"), "001" ("string")) -> (w8801:string)
            n4982 = String To Byte Array(string=w8801) -> (unsigned byte array=w8806:u8[])
            n4983 = for {
              tunnel: w8806 -> [w8827] mode=indexing
              shift-right: [w8825] -> w8808
              shift-left: u8 0 -> [w8826]
              n4984 = Add(x=w8827, y=w8826) -> (x+y=w8825:u8)
            }
            n4985 = Number To Decimal String(number=w8808) -> (decimal integer string=w8803:string)  [unwired: 1 in]
            n4986 = String Length(string=w8803) -> (length=w8804:i32)
            n4987 = case shown="0, Default" w8804 {
              tunnel: w8803 -> [_ w8820 w8823 w8824]
              tunnel: ["" w8818 w8821 w8824] -> w8802
              frame 0, Default {
              }
              frame 1 {
                n4988 = Concatenate Strings("00" ("string"), w8820) -> (w8818:string)
              }
              frame 2 {
                n4989 = Concatenate Strings("0" ("string"), w8823) -> (w8821:string)
              }
              frame 3 {
              }
            }
            n4990 = local write "Tp2 auto low speed"(FALSE ("Tp2_auto_low_speed")) -> ()
            n4991 = Concatenate Strings(w8801, w8802, "\r") -> (w8798:string)
            n4992 = VISA Write(VISA resource name=w8797, write buffer=w8798, error in (no error)=w8796) -> (VISA resource name out=w8800:refnum<visa-resource-name>, error out=w8799:errorcluster)  [unwired: 1 out]
            n4993 = stacked-sequence {
              tunnel: [w8816] -> w8795
              tunnel: w8800 -> [w8816]
              tunnel: [w8815] -> w8794
              tunnel: w8799 -> [w8815]
              frame #0 {
                n4994 = Wait (ms)(milliseconds to wait=u32 100) -> ()  [unwired: 1 out]
              }
            }
          }
          frame 5 {
            # "Address"
            n4995 = Concatenate Strings("001" ("write buffer"), "10" ("string"), "026" ("string"), "03" ("string"), "000" ("string")) -> (w8836:string)
            n4996 = String To Byte Array(string=w8836) -> (unsigned byte array=w8841:u8[])
            n4997 = for {
              tunnel: w8841 -> [w8862] mode=indexing
              shift-right: [w8860] -> w8843
              shift-left: u8 0 -> [w8861]
              n4998 = Add(x=w8862, y=w8861) -> (x+y=w8860:u8)
            }
            n4999 = Number To Decimal String(number=w8843) -> (decimal integer string=w8838:string)  [unwired: 1 in]
            n5000 = String Length(string=w8838) -> (length=w8839:i32)
            n5001 = local write "Tp2 auto normal speed"(FALSE ("Tp2_auto_normal_speed")) -> ()
            n5002 = case shown="0, Default" w8839 {
              tunnel: w8838 -> [_ w8855 w8858 w8859]
              tunnel: ["" w8853 w8856 w8859] -> w8837
              frame 0, Default {
              }
              frame 1 {
                n5003 = Concatenate Strings("00" ("string"), w8855) -> (w8853:string)
              }
              frame 2 {
                n5004 = Concatenate Strings("0" ("string"), w8858) -> (w8856:string)
              }
              frame 3 {
              }
            }
            n5005 = Concatenate Strings(w8836, w8837, "\r") -> (w8833:string)
            n5006 = VISA Write(VISA resource name=w8832, write buffer=w8833, error in (no error)=w8831) -> (VISA resource name out=w8835:refnum<visa-resource-name>, error out=w8834:errorcluster)  [unwired: 1 out]
            n5007 = stacked-sequence {
              tunnel: [w8851] -> w8830
              tunnel: w8835 -> [w8851]
              tunnel: [w8850] -> w8829
              tunnel: w8834 -> [w8850]
              frame #0 {
                n5008 = Wait (ms)(milliseconds to wait=u32 100) -> ()  [unwired: 1 out]
              }
            }
          }
          frame 6 {
            # "Cheksum 3 haneli olmalı"
            # "Address"
            n5009 = Concatenate Strings("001" ("write buffer"), "10" ("string"), "023" ("string"), "06" ("string"), "111111" ("string")) -> (w8870:string)
            n5010 = String To Byte Array(string=w8870) -> (unsigned byte array=w8875:u8[])
            n5011 = for {
              tunnel: w8875 -> [w8896] mode=indexing
              shift-right: [w8894] -> w8877
              shift-left: u8 0 -> [w8895]
              n5012 = Add(x=w8896, y=w8895) -> (x+y=w8894:u8)
            }
            n5013 = Number To Decimal String(number=w8877) -> (decimal integer string=w8872:string)  [unwired: 1 in]
            n5014 = String Length(string=w8872) -> (length=w8873:i32)
            n5015 = case shown="0, Default" w8873 {
              tunnel: w8872 -> [_ w8889 w8892 w8893]
              tunnel: ["" w8887 w8890 w8893] -> w8871
              frame 0, Default {
              }
              frame 1 {
                n5016 = Concatenate Strings("00" ("string"), w8889) -> (w8887:string)
              }
              frame 2 {
                n5017 = Concatenate Strings("0" ("string"), w8892) -> (w8890:string)
              }
              frame 3 {
              }
            }
            n5018 = Concatenate Strings(w8870, w8871, "\r") -> (w8867:string)
            n5019 = VISA Write(VISA resource name=w8866, write buffer=w8867, error in (no error)=w8865) -> (VISA resource name out=w8869:refnum<visa-resource-name>, error out=w8868:errorcluster)  [unwired: 1 out]
            n5020 = stacked-sequence {
              tunnel: [w8885] -> w8864
              tunnel: w8869 -> [w8885]
              tunnel: [w8884] -> w8863
              tunnel: w8868 -> [w8884]
              frame #0 {
                n5021 = Wait (ms)(milliseconds to wait=u32 100) -> ()  [unwired: 1 out]
              }
            }
          }
          frame 7 {
            # "Cheksum 3 haneli olmalı"
            # "Address"
            n5022 = Concatenate Strings("001" ("write buffer"), "10" ("string"), "023" ("string"), "06" ("string"), "000000" ("string")) -> (w8904:string)
            n5023 = String To Byte Array(string=w8904) -> (unsigned byte array=w8909:u8[])
            n5024 = for {
              tunnel: w8909 -> [w8930] mode=indexing
              shift-right: [w8928] -> w8911
              shift-left: u8 0 -> [w8929]
              n5025 = Add(x=w8930, y=w8929) -> (x+y=w8928:u8)
            }
            n5026 = Number To Decimal String(number=w8911) -> (decimal integer string=w8906:string)  [unwired: 1 in]
            n5027 = String Length(string=w8906) -> (length=w8907:i32)
            n5028 = case shown="0, Default" w8907 {
              tunnel: w8906 -> [_ w8923 w8926 w8927]
              tunnel: ["" w8921 w8924 w8927] -> w8905
              frame 0, Default {
              }
              frame 1 {
                n5029 = Concatenate Strings("00" ("string"), w8923) -> (w8921:string)
              }
              frame 2 {
                n5030 = Concatenate Strings("0" ("string"), w8926) -> (w8924:string)
              }
              frame 3 {
              }
            }
            n5031 = Concatenate Strings(w8904, w8905, "\r") -> (w8901:string)
            n5032 = VISA Write(VISA resource name=w8900, write buffer=w8901, error in (no error)=w8899) -> (VISA resource name out=w8903:refnum<visa-resource-name>, error out=w8902:errorcluster)  [unwired: 1 out]
            n5033 = stacked-sequence {
              tunnel: [w8919] -> w8898
              tunnel: w8903 -> [w8919]
              tunnel: [w8918] -> w8897
              tunnel: w8902 -> [w8918]
              frame #0 {
                n5034 = Wait (ms)(milliseconds to wait=u32 100) -> ()  [unwired: 1 out]
              }
            }
          }
        }
      }
      frame #2 {
        n5035 = Or(x="Tp3 set speed gui", y="Tp3 auto set speed") -> (x .or. y?=w8954:bool)
        n5036 = Compound Arithmetic op=OR("Tp3 start gui", "Tp3 start gui 1", "Tp3 auto start") -> (w8936:bool)
        n5037 = Compound Arithmetic op=OR("Tp3 stop gui", "Tp3 stop gui 1", "Tp3 auto stop") -> (w8939:bool)
        n5038 = Or(x="Tp3 low speed gui", y="Tp3 auto low speed") -> (x .or. y?=w8937:bool)
        n5039 = Or(x="Tp3 normal speed gui", y="Tp3 auto normal speed") -> (x .or. y?=w8949:bool)
        n5040 = case shown="True" w8936 {
          tunnel: [FALSE w8962] -> w8935
          frame False {
          }
          frame True {
            n5041 = case shown="True" "tp3 start safety" {
              tunnel: [FALSE TRUE] -> w8962
              frame False {
                n5042 = local write "Tp3 auto start"(FALSE ("Tp1_auto_start")) -> ()
                n5043 = local write "Warning Message"("CH3 TP cannot be started." ("Error Message")) -> ()
              }
              frame True {
              }
            }
          }
        }
        n5044 = Build Array(FALSE, w8935, w8939, w8954, w8937, w8949, "Tp3 start initial", "Tp3 stop initial", "Adress set") -> (w8946:bool[])
        n5045 = Boolean Array To Number(Boolean array=w8946) -> (number=w8959:u32)
        n5046 = Mantissa & Exponent(0:w8959) -> (2:w8958:dbl)  [unwired: 1 out]
        n5047 = case shown="0, Default" w8958 {
          tunnel: w8934 -> [w8969 w9082 w9118 w9160 w9203 w9238 w9272 w9306]
          tunnel: w8933 -> [w8970 w9081 w9117 w9159 w9202 w9237 w9271 w9305]
          tunnel: [w8968 w9079 w9114 w9151 w9201 w9236 w9270 w9304] -> w8932
          tunnel: [w8967 w9078 w9113 w9150 w9200 w9235 w9269 w9303] -> w8931
          frame 0, Default {
            n5048 = stacked-sequence {
              seq-local: [w8976 _] -> [_ w9034]
              seq-local: [w8975 _] -> [_ w9035]
              tunnel: w8969 -> [w8986 _]
              tunnel: w8970 -> [w8985 _]
              tunnel: [_ w9037] -> w8968
              tunnel: [_ w9036] -> w8967
              frame #0 {
                # "Address"
                # "Cheksum 3 haneli olmalı"
                # "Address"
                n5049 = Concatenate Strings("003" ("write buffer"), "00" ("string"), "309" ("string"), "02" ("string"), "=?" ("string")) -> (w8995:string)
                n5050 = String To Byte Array(string=w8995) -> (unsigned byte array=w9000:u8[])
                n5051 = for {
                  tunnel: w9000 -> [w9032] mode=indexing
                  shift-right: [w9030] -> w9002
                  shift-left: u8 0 -> [w9031]
                  n5052 = Add(x=w9032, y=w9031) -> (x+y=w9030:u8)
                }
                n5053 = Number To Decimal String(number=w9002) -> (decimal integer string=w8997:string)  [unwired: 1 in]
                n5054 = String Length(string=w8997) -> (length=w8998:i32)
                n5055 = case shown="0, Default" w8998 {
                  tunnel: w8997 -> [_ w9025 w9028 w9029]
                  tunnel: ["" w9023 w9026 w9029] -> w8996
                  frame 0, Default {
                  }
                  frame 1 {
                    n5056 = Concatenate Strings("00" ("string"), w9025) -> (w9023:string)
                  }
                  frame 2 {
                    n5057 = Concatenate Strings("0" ("string"), w9028) -> (w9026:string)
                  }
                  frame 3 {
                  }
                }
                n5058 = Concatenate Strings(w8995, w8996, "\r") -> (w8987:string)
                n5059 = VISA Write(VISA resource name=w8986, write buffer=w8987, error in (no error)=w8985) -> (VISA resource name out=w8990:refnum<visa-resource-name>, error out=w8989:errorcluster)  [unwired: 1 out]
                n5060 = stacked-sequence {
                  tunnel: [w9021] -> w8992
                  tunnel: w8990 -> [w9021]
                  tunnel: [w9020] -> w8991
                  tunnel: w8989 -> [w9020]
                  frame #0 {
                    n5061 = Wait (ms)(milliseconds to wait=u32 100) -> ()  [unwired: 1 out]
                  }
                }
                n5062 = property class="Instr"(reference=w8992, error in=w8991) -> (reference out=w8994:refnum<visa-resource-name>, error out=w8993:errorcluster, "Serial Settings:Number of Bytes at Serial Port"=w8988:u32)
                n5063 = VISA Read(VISA resource name=w8994, byte count=w8988, error in (no error)=w8993) -> (VISA resource name out=w8976:refnum<visa-resource-name>, read buffer=w8983:string, error out=w8975:errorcluster)  [unwired: 1 out]
                n5064 = String Length(string=w8983) -> (length=w8984:i32)
                n5065 = Not Equal To 0?(x=w8984) -> (x != 0?=w8974:bool)
                n5066 = feedback #144() -> (w8971:bool)  [unwired: 1 in]
                n5067 = Concatenate Strings("003" ("regular expression"), "1030906" ("regular expression")) -> (w8982:string)
                n5068 = Match Pattern(string=w8983, regular expression=w8982) -> (after substring=w8977:string)  [unwired: 4 out]
                n5069 = case shown="False" w8974 {
                  tunnel: [FALSE w9012] -> w8973
                  tunnel: [TRUE FALSE] -> w8972
                  tunnel: w8971 -> [_ w9010]
                  frame False {
                  }
                  frame True {
                    n5070 = call "Elapsed Time39"("Reset"=w9010) -> ("Elapsed Time (s)"=w9013:dbl)  [unwired: 11 in, 7 out]
                    n5071 = Greater?(x=w9013, y=5.0) -> (0:w9012:bool)
                  }
                }
                "tp3 com" <- w8973
                n5072 = feedback-in #144(w8972) -> ()
                n5073 = String Length(string=w8977) -> (length=w8979:i32)
                n5074 = Not Equal To 0?(x=w8979) -> (x != 0?=w8978:bool)
                n5075 = case shown="True" w8978 {
                  tunnel: w8977 -> [_ w9016]
                  frame False {
                  }
                  frame True {
                    n5076 = String Subset(string=w9016, length (rest)=6 ("length (rest)")) -> (substring=w9017:string)  [unwired: 1 out]
                    n5077 = Decimal String To Number(string=w9017) -> (number=→"Tp3 speed gui":i32)  [unwired: 3 out]
                    "tp3 readout" <- w9016
                  }
                }
              }
              frame #1 {
                # "Address"
                # "Cheksum 3 haneli olmalı"
                # "Address"
                n5078 = Concatenate Strings("003" ("write buffer"), "00" ("string"), "307" ("string"), "02" ("string"), "=?" ("string")) -> (w9050:string)
                n5079 = String To Byte Array(string=w9050) -> (unsigned byte array=w9055:u8[])
                n5080 = for {
                  tunnel: w9055 -> [w9076] mode=indexing
                  shift-right: [w9074] -> w9057
                  shift-left: u8 0 -> [w9075]
                  n5081 = Add(x=w9076, y=w9075) -> (x+y=w9074:u8)
                }
                n5082 = Number To Decimal String(number=w9057) -> (decimal integer string=w9052:string)  [unwired: 1 in]
                n5083 = String Length(string=w9052) -> (length=w9053:i32)
                n5084 = case shown="0, Default" w9053 {
                  tunnel: w9052 -> [_ w9069 w9072 w9073]
                  tunnel: ["" w9067 w9070 w9073] -> w9051
                  frame 0, Default {
                  }
                  frame 1 {
                    n5085 = Concatenate Strings("00" ("string"), w9069) -> (w9067:string)
                  }
                  frame 2 {
                    n5086 = Concatenate Strings("0" ("string"), w9072) -> (w9070:string)
                  }
                  frame 3 {
                  }
                }
                n5087 = Concatenate Strings(w9050, w9051, "\r") -> (w9042:string)
                n5088 = VISA Write(VISA resource name=w9034, write buffer=w9042, error in (no error)=w9035) -> (VISA resource name out=w9045:refnum<visa-resource-name>, error out=w9044:errorcluster)  [unwired: 1 out]
                n5089 = stacked-sequence {
                  tunnel: [w9065] -> w9047
                  tunnel: w9045 -> [w9065]
                  tunnel: [w9064] -> w9046
                  tunnel: w9044 -> [w9064]
                  frame #0 {
                    n5090 = Wait (ms)(milliseconds to wait=u32 100) -> ()  [unwired: 1 out]
                  }
                }
                n5091 = property class="Instr"(reference=w9047, error in=w9046) -> (reference out=w9049:refnum<visa-resource-name>, error out=w9048:errorcluster, "Serial Settings:Number of Bytes at Serial Port"=w9043:u32)
                n5092 = VISA Read(VISA resource name=w9049, byte count=w9043, error in (no error)=w9048) -> (VISA resource name out=w9037:refnum<visa-resource-name>, read buffer=w9041:string, error out=w9036:errorcluster)  [unwired: 1 out]
                n5093 = Concatenate Strings("003" ("regular expression"), "1030706" ("regular expression")) -> (w9040:string)
                n5094 = Match Pattern(string=w9041, regular expression=w9040) -> (after substring=→"after substring 3":string)  [unwired: 4 out]
              }
            }
          }
          frame 1 {
            # "Address"
            n5095 = Concatenate Strings("003" ("write buffer"), "10" ("string"), "010" ("string"), "06" ("string"), "111111" ("string")) -> (w9086:string)
            n5096 = String To Byte Array(string=w9086) -> (unsigned byte array=w9091:u8[])
            n5097 = for {
              tunnel: w9091 -> [w9112] mode=indexing
              shift-right: [w9110] -> w9093
              shift-left: u8 0 -> [w9111]
              n5098 = Add(x=w9112, y=w9111) -> (x+y=w9110:u8)
            }
            n5099 = Number To Decimal String(number=w9093) -> (decimal integer string=w9088:string)  [unwired: 1 in]
            n5100 = String Length(string=w9088) -> (length=w9089:i32)
            n5101 = local write "Tp3 auto start"(FALSE ("Tp3_auto_start")) -> ()
            n5102 = case shown="0, Default" w9089 {
              tunnel: w9088 -> [_ w9105 w9108 w9109]
              tunnel: ["" w9103 w9106 w9109] -> w9087
              frame 0, Default {
              }
              frame 1 {
                n5103 = Concatenate Strings("00" ("string"), w9105) -> (w9103:string)
              }
              frame 2 {
                n5104 = Concatenate Strings("0" ("string"), w9108) -> (w9106:string)
              }
              frame 3 {
              }
            }
            n5105 = local write "Tp3_stop_cmnd"(FALSE ("Tp3_auto_start")) -> ()
            n5106 = Concatenate Strings(w9086, w9087, "\r") -> (w9083:string)
            n5107 = VISA Write(VISA resource name=w9082, write buffer=w9083, error in (no error)=w9081) -> (VISA resource name out=w9085:refnum<visa-resource-name>, error out=w9084:errorcluster)  [unwired: 1 out]
            n5108 = stacked-sequence {
              tunnel: [w9101] -> w9079
              tunnel: w9085 -> [w9101]
              tunnel: [w9100] -> w9078
              tunnel: w9084 -> [w9100]
              frame #0 {
                n5109 = Wait (ms)(milliseconds to wait=u32 100) -> ()  [unwired: 1 out]
              }
            }
          }
          frame 2 {